vi "Dresden R2R Sputter 03.02.2018 IY24.vi"() -> ()   [LabVIEW 2009] (continued)
              shift-right: [w14079] -> w14054
              shift-left: i16? 0 -> [w14080]
              n8824 = Add(x=w14081, y=w14080) -> (x+y=w14079)
            }
            n8825 = Number To Decimal String(number=w14054) -> (decimal integer string=w14049)  [unwired: 1 in]
            n8826 = String Length(string=w14049) -> (length=w14050)
            n8827 = case shown="0, Default" w14050 {
              tunnel: w14049 -> [_ w14074 w14077 w14078]
              tunnel: [data[5B] w14072 w14075 w14078] -> w14048
              frame #0 {
              }
              frame #1 {
                n8828 = Concatenate Strings("00" ("string"), w14074) -> (w14072)
              }
              frame #2 {
                n8829 = Concatenate Strings("0" ("string"), w14077) -> (w14075)
              }
              frame #3 {
              }
            }
            n8830 = Concatenate Strings(w14047, w14048, "\n") -> (w14044)
            n8831 = VISA Write(VISA resource name=w14043, write buffer=w14044, error in (no error)=w14042) -> (VISA resource name out=w14046, error out=w14045)  [unwired: 1 out]
            n8832 = stacked-sequence {
              tunnel: [w14070] -> w14041
              tunnel: w14046 -> [w14070]
              tunnel: [w14069] -> w14040
              tunnel: w14045 -> [w14069]
              frame #0 {
                n8833 = Wait (ms)(milliseconds to wait=i32? 100) -> ()  [unwired: 1 out]
              }
            }
          }
          frame #4 {
            # "Cheksum 3 haneli olmalı"
            # "Address"
            n8834 = Concatenate Strings("002" ("write buffer"), "10" ("string"), "026" ("string"), "03" ("string"), "001" ("string")) -> (w14089)
            n8835 = String To Byte Array(string=w14089) -> (unsigned byte array=w14094)
            n8836 = for {
              tunnel: w14094 -> [w14115] mode=indexing
              shift-right: [w14113] -> w14096
              shift-left: i16? 0 -> [w14114]
              n8837 = Add(x=w14115, y=w14114) -> (x+y=w14113)
            }
            n8838 = Number To Decimal String(number=w14096) -> (decimal integer string=w14091)  [unwired: 1 in]
            n8839 = String Length(string=w14091) -> (length=w14092)
            n8840 = case shown="0, Default" w14092 {
              tunnel: w14091 -> [_ w14108 w14111 w14112]
              tunnel: [data[5B] w14106 w14109 w14112] -> w14090
              frame #0 {
              }
              frame #1 {
                n8841 = Concatenate Strings("00" ("string"), w14108) -> (w14106)
              }
              frame #2 {
                n8842 = Concatenate Strings("0" ("string"), w14111) -> (w14109)
              }
              frame #3 {
              }
            }
            n8843 = Concatenate Strings(w14089, w14090, "\n") -> (w14086)
            n8844 = VISA Write(VISA resource name=w14085, write buffer=w14086, error in (no error)=w14084) -> (VISA resource name out=w14088, error out=w14087)  [unwired: 1 out]
            n8845 = stacked-sequence {
              tunnel: [w14104] -> w14083
              tunnel: w14088 -> [w14104]
              tunnel: [w14103] -> w14082
              tunnel: w14087 -> [w14103]
              frame #0 {
                n8846 = Wait (ms)(milliseconds to wait=i32? 100) -> ()  [unwired: 1 out]
              }
            }
          }
          frame #5 {
            # "Address"
            n8847 = Concatenate Strings("002" ("write buffer"), "10" ("string"), "026" ("string"), "03" ("string"), "000" ("string")) -> (w14123)
            n8848 = String To Byte Array(string=w14123) -> (unsigned byte array=w14128)
            n8849 = for {
              tunnel: w14128 -> [w14149] mode=indexing
              shift-right: [w14147] -> w14130
              shift-left: i16? 0 -> [w14148]
              n8850 = Add(x=w14149, y=w14148) -> (x+y=w14147)
            }
            n8851 = Number To Decimal String(number=w14130) -> (decimal integer string=w14125)  [unwired: 1 in]
            n8852 = String Length(string=w14125) -> (length=w14126)
            n8853 = case shown="0, Default" w14126 {
              tunnel: w14125 -> [_ w14142 w14145 w14146]
              tunnel: [data[5B] w14140 w14143 w14146] -> w14124
              frame #0 {
              }
              frame #1 {
                n8854 = Concatenate Strings("00" ("string"), w14142) -> (w14140)
              }
              frame #2 {
                n8855 = Concatenate Strings("0" ("string"), w14145) -> (w14143)
              }
              frame #3 {
              }
            }
            n8856 = Concatenate Strings(w14123, w14124, "\n") -> (w14120)
            n8857 = VISA Write(VISA resource name=w14119, write buffer=w14120, error in (no error)=w14118) -> (VISA resource name out=w14122, error out=w14121)  [unwired: 1 out]
            n8858 = stacked-sequence {
              tunnel: [w14138] -> w14117
              tunnel: w14122 -> [w14138]
              tunnel: [w14137] -> w14116
              tunnel: w14121 -> [w14137]
              frame #0 {
                n8859 = Wait (ms)(milliseconds to wait=i32? 100) -> ()  [unwired: 1 out]
              }
            }
          }
          frame #6 {
            # "Cheksum 3 haneli olmalı"
            # "Address"
            n8860 = Concatenate Strings("002" ("write buffer"), "10" ("string"), "023" ("string"), "06" ("string"), "111111" ("string")) -> (w14157)
            n8861 = String To Byte Array(string=w14157) -> (unsigned byte array=w14162)
            n8862 = for {
              tunnel: w14162 -> [w14183] mode=indexing
              shift-right: [w14181] -> w14164
              shift-left: i16? 0 -> [w14182]
              n8863 = Add(x=w14183, y=w14182) -> (x+y=w14181)
            }
            n8864 = Number To Decimal String(number=w14164) -> (decimal integer string=w14159)  [unwired: 1 in]
            n8865 = String Length(string=w14159) -> (length=w14160)
            n8866 = case shown="0, Default" w14160 {
              tunnel: w14159 -> [_ w14176 w14179 w14180]
              tunnel: [data[5B] w14174 w14177 w14180] -> w14158
              frame #0 {
              }
              frame #1 {
                n8867 = Concatenate Strings("00" ("string"), w14176) -> (w14174)
              }
              frame #2 {
                n8868 = Concatenate Strings("0" ("string"), w14179) -> (w14177)
              }
              frame #3 {
              }
            }
            n8869 = Concatenate Strings(w14157, w14158, "\n") -> (w14154)
            n8870 = VISA Write(VISA resource name=w14153, write buffer=w14154, error in (no error)=w14152) -> (VISA resource name out=w14156, error out=w14155)  [unwired: 1 out]
            n8871 = stacked-sequence {
              tunnel: [w14172] -> w14151
              tunnel: w14156 -> [w14172]
              tunnel: [w14171] -> w14150
              tunnel: w14155 -> [w14171]
              frame #0 {
                n8872 = Wait (ms)(milliseconds to wait=i32? 100) -> ()  [unwired: 1 out]
              }
            }
          }
          frame #7 {
            # "Cheksum 3 haneli olmalı"
            # "Address"
            n8873 = Concatenate Strings("002" ("write buffer"), "10" ("string"), "023" ("string"), "06" ("string"), "000000" ("string")) -> (w14191)
            n8874 = String To Byte Array(string=w14191) -> (unsigned byte array=w14196)
            n8875 = for {
              tunnel: w14196 -> [w14217] mode=indexing
              shift-right: [w14215] -> w14198
              shift-left: i16? 0 -> [w14216]
              n8876 = Add(x=w14217, y=w14216) -> (x+y=w14215)
            }
            n8877 = Number To Decimal String(number=w14198) -> (decimal integer string=w14193)  [unwired: 1 in]
            n8878 = String Length(string=w14193) -> (length=w14194)
            n8879 = case shown="0, Default" w14194 {
              tunnel: w14193 -> [_ w14210 w14213 w14214]
              tunnel: [data[5B] w14208 w14211 w14214] -> w14192
              frame #0 {
              }
              frame #1 {
                n8880 = Concatenate Strings("00" ("string"), w14210) -> (w14208)
              }
              frame #2 {
                n8881 = Concatenate Strings("0" ("string"), w14213) -> (w14211)
              }
              frame #3 {
              }
            }
            n8882 = Concatenate Strings(w14191, w14192, "\n") -> (w14188)
            n8883 = VISA Write(VISA resource name=w14187, write buffer=w14188, error in (no error)=w14186) -> (VISA resource name out=w14190, error out=w14189)  [unwired: 1 out]
            n8884 = stacked-sequence {
              tunnel: [w14206] -> w14185
              tunnel: w14190 -> [w14206]
              tunnel: [w14205] -> w14184
              tunnel: w14189 -> [w14205]
              frame #0 {
                n8885 = Wait (ms)(milliseconds to wait=i32? 100) -> ()  [unwired: 1 out]
              }
            }
          }
        }
      }
      frame #2 {
        n8886 = Or(x="Set_speed Tp3", y="Tp3_auto_set_speed") -> (x .or. y?=w14241)
        n8887 = Compound Arithmetic op=OR("Start Tp3", "Tp_start_ch3_gui", "Tp3_auto_start") -> (w14223)
        n8888 = Compound Arithmetic op=OR("Stop Tp3", "Tp_stop_ch3_gui", "Tp3_auto_stop") -> (w14226)
        n8889 = Or(x="Low_speed Tp3", y="Tp3_auto_low_speed") -> (x .or. y?=w14224)
        n8890 = Or(x="Normal_speed Tp3", y="Tp3_auto_normal_speed") -> (x .or. y?=w14236)
        n8891 = case shown="False" w14223 {
          tunnel: [i16? 0 w14248] -> w14222
          frame #0 {
          }
          frame #1 {
            n8892 = local read "Ch3_Tp_start_safety"() -> (w14249)
            n8893 = case shown="True" w14249 {
              tunnel: [i16? 0 T/1] -> w14248
              frame #0 {
                n8894 = local write "Tp3_auto_start"(i16? 0 ("Tp1_auto_start")) -> ()
                n8895 = local write "Error Message"("TP can not be started.\nReason:\n*MP can not be open                           *TP-BV can not be open.       *Pressure difference                                between chamber and pipeline \nnot suitable.\n                                      \n" ("Error Message")) -> ()
              }
              frame #1 {
              }
            }
          }
        }
        n8896 = Build Array(i16? 0, w14222, w14226, w14241, w14224, w14236, "Start_initial Tp3", "Stop_initial Tp3", "Adress set") -> (w14233)
        n8897 = Boolean Array To Number(Boolean array=w14233) -> (number=w14246)
        n8898 = Mantissa & Exponent(0:w14246) -> (2:w14245)  [unwired: 1 out]
        n8899 = case shown="0, Default" w14245 {
          tunnel: w14221 -> [w14256 w14369 w14405 w14446 w14488 w14522 w14556 w14590]
          tunnel: w14220 -> [w14257 w14368 w14404 w14445 w14487 w14521 w14555 w14589]
          tunnel: [w14255 w14366 w14401 w14437 w14486 w14520 w14554 w14588] -> w14219
          tunnel: [w14254 w14365 w14400 w14436 w14485 w14519 w14553 w14587] -> w14218
          frame #0 {
            n8900 = stacked-sequence {
              tunnel: w14256 -> [w14273 _]
              tunnel: w14257 -> [w14272 _]
              tunnel: [_ w14324] -> w14255
              tunnel: [_ w14323] -> w14254
              frame #0 {
                # "Address"
                # "Cheksum 3 haneli olmalı"
                # "Address"
                n8901 = Concatenate Strings("003" ("write buffer"), "00" ("string"), "309" ("string"), "02" ("string"), "=?" ("string")) -> (w14282)
                n8902 = String To Byte Array(string=w14282) -> (unsigned byte array=w14287)
                n8903 = for {
                  tunnel: w14287 -> [w14319] mode=indexing
                  shift-right: [w14317] -> w14289
                  shift-left: i16? 0 -> [w14318]
                  n8904 = Add(x=w14319, y=w14318) -> (x+y=w14317)
                }
                n8905 = Number To Decimal String(number=w14289) -> (decimal integer string=w14284)  [unwired: 1 in]
                n8906 = String Length(string=w14284) -> (length=w14285)
                n8907 = case shown="0, Default" w14285 {
                  tunnel: w14284 -> [_ w14312 w14315 w14316]
                  tunnel: [data[5B] w14310 w14313 w14316] -> w14283
                  frame #0 {
                  }
                  frame #1 {
                    n8908 = Concatenate Strings("00" ("string"), w14312) -> (w14310)
                  }
                  frame #2 {
                    n8909 = Concatenate Strings("0" ("string"), w14315) -> (w14313)
                  }
                  frame #3 {
                  }
                }
                n8910 = Concatenate Strings(w14282, w14283, "\n") -> (w14274)
                n8911 = VISA Write(VISA resource name=w14273, write buffer=w14274, error in (no error)=w14272) -> (VISA resource name out=w14277, error out=w14276)  [unwired: 1 out]
                n8912 = stacked-sequence {
                  tunnel: [w14308] -> w14279
                  tunnel: w14277 -> [w14308]
                  tunnel: [w14307] -> w14278
                  tunnel: w14276 -> [w14307]
                  frame #0 {
                    n8913 = Wait (ms)(milliseconds to wait=i32? 100) -> ()  [unwired: 1 out]
                  }
                }
                n8914 = property class="Instr"(reference=w14279, error in=w14278) -> (reference out=w14281, error out=w14280, "Serial Settings:Number of Bytes at Serial Port"=w14275)
                n8915 = VISA Read(VISA resource name=w14281, byte count=w14275, error in (no error)=w14280) -> (VISA resource name out=w14263, read buffer=w14270, error out=w14262)  [unwired: 1 out]
                "Read_data 6" <- w14270
                n8916 = String Length(string=w14270) -> (length=w14271)
                n8917 = Not Equal To 0?(x=w14271) -> (x != 0?=w14261)
                n8918 = feedback #279() -> (w14258)  [unwired: 1 in]
                n8919 = Concatenate Strings("003" ("regular expression"), "1030906" ("regular expression")) -> (w14269)
                n8920 = Match Pattern(string=w14270, regular expression=w14269) -> (after substring=w14264)  [unwired: 4 out]
                n8921 = case shown="True" w14261 {
                  tunnel: [i16? 0 w14299] -> w14260
                  tunnel: [T/1 i16? 0] -> w14259
                  tunnel: w14258 -> [_ w14297]
                  frame #0 {
                  }
                  frame #1 {
                    n8922 = call "Elapsed Time133"(2:w14297) -> (16:w14300)  [unwired: 11 in, 7 out]
                    n8923 = Greater?(x=w14300, y=dbl? 5.0) -> (0:w14299)
                  }
                }
                "Com_ok 3" <- w14260
                n8924 = String Length(string=w14264) -> (length=w14266)
                n8925 = Not Equal To 0?(x=w14266) -> (x != 0?=w14265)
                n8926 = case shown="True" w14265 {
                  tunnel: w14264 -> [_ w14303]
                  frame #0 {
                  }
                  frame #1 {
                    n8927 = String Subset(string=w14303, length (rest)=i32? 6 ("length (rest)")) -> (substring=w14304)  [unwired: 1 out]
                    n8928 = Decimal String To Number(string=w14304) -> (number=→"Tp3_speed_gui" →"Turbo_pump_speed 5")  [unwired: 3 out]
                  }
                }
              }
              frame #1 {
                # "Address"
                # "Cheksum 3 haneli olmalı"
                # "Address"
                n8929 = Concatenate Strings("003" ("write buffer"), "00" ("string"), "307" ("string"), "02" ("string"), "=?" ("string")) -> (w14337)
                n8930 = String To Byte Array(string=w14337) -> (unsigned byte array=w14342)
                n8931 = for {
                  tunnel: w14342 -> [w14363] mode=indexing
                  shift-right: [w14361] -> w14344
                  shift-left: i16? 0 -> [w14362]
                  n8932 = Add(x=w14363, y=w14362) -> (x+y=w14361)
                }
                n8933 = Number To Decimal String(number=w14344) -> (decimal integer string=w14339)  [unwired: 1 in]
                n8934 = String Length(string=w14339) -> (length=w14340)
                n8935 = case shown="0, Default" w14340 {
                  tunnel: w14339 -> [_ w14356 w14359 w14360]
                  tunnel: [data[5B] w14354 w14357 w14360] -> w14338
                  frame #0 {
                  }
                  frame #1 {
                    n8936 = Concatenate Strings("00" ("string"), w14356) -> (w14354)
                  }
                  frame #2 {
                    n8937 = Concatenate Strings("0" ("string"), w14359) -> (w14357)
                  }
                  frame #3 {
                  }
                }
                n8938 = Concatenate Strings(w14337, w14338, "\n") -> (w14329)
                n8939 = VISA Write(VISA resource name=w14321, write buffer=w14329, error in (no error)=w14322) -> (VISA resource name out=w14332, error out=w14331)  [unwired: 1 out]
                n8940 = stacked-sequence {
                  tunnel: [w14352] -> w14334
                  tunnel: w14332 -> [w14352]
                  tunnel: [w14351] -> w14333
                  tunnel: w14331 -> [w14351]
                  frame #0 {
                    n8941 = Wait (ms)(milliseconds to wait=i32? 100) -> ()  [unwired: 1 out]
                  }
                }
                n8942 = property class="Instr"(reference=w14334, error in=w14333) -> (reference out=w14336, error out=w14335, "Serial Settings:Number of Bytes at Serial Port"=w14330)
                n8943 = VISA Read(VISA resource name=w14336, byte count=w14330, error in (no error)=w14335) -> (VISA resource name out=w14324, read buffer=w14328, error out=w14323)  [unwired: 1 out]
                "Read_data 7" <- w14328
                n8944 = Concatenate Strings("003" ("regular expression"), "1030706" ("regular expression")) -> (w14327)
                n8945 = Match Pattern(string=w14328, regular expression=w14327) -> (after substring=→"after substring 3")  [unwired: 4 out]
              }
            }
          }
          frame #1 {
            # "Address"
            n8946 = Concatenate Strings("003" ("write buffer"), "10" ("string"), "010" ("string"), "06" ("string"), "111111" ("string")) -> (w14373)
            n8947 = String To Byte Array(string=w14373) -> (unsigned byte array=w14378)
            n8948 = for {
              tunnel: w14378 -> [w14399] mode=indexing
              shift-right: [w14397] -> w14380
              shift-left: i16? 0 -> [w14398]
              n8949 = Add(x=w14399, y=w14398) -> (x+y=w14397)
            }
            n8950 = Number To Decimal String(number=w14380) -> (decimal integer string=w14375)  [unwired: 1 in]
            n8951 = String Length(string=w14375) -> (length=w14376)
            n8952 = local write "Tp3_auto_start"(i16? 0 ("Tp3_auto_start")) -> ()
            n8953 = case shown="0, Default" w14376 {
              tunnel: w14375 -> [_ w14392 w14395 w14396]
              tunnel: [data[5B] w14390 w14393 w14396] -> w14374
              frame #0 {
              }
              frame #1 {
                n8954 = Concatenate Strings("00" ("string"), w14392) -> (w14390)
              }
              frame #2 {
                n8955 = Concatenate Strings("0" ("string"), w14395) -> (w14393)
              }
              frame #3 {
              }
            }
            n8956 = local write "Tp3_stop_cmnd"(i16? 0 ("Tp3_auto_start")) -> ()
            n8957 = Concatenate Strings(w14373, w14374, "\n") -> (w14370)
            n8958 = VISA Write(VISA resource name=w14369, write buffer=w14370, error in (no error)=w14368) -> (VISA resource name out=w14372, error out=w14371)  [unwired: 1 out]
            n8959 = stacked-sequence {
              tunnel: [w14388] -> w14366
              tunnel: w14372 -> [w14388]
              tunnel: [w14387] -> w14365
              tunnel: w14371 -> [w14387]
              frame #0 {
                n8960 = Wait (ms)(milliseconds to wait=i32? 100) -> ()  [unwired: 1 out]
              }
            }
          }
          frame #2 {
            # "Cheksum 3 haneli olmalı"
            # "Address"
            n8961 = Concatenate Strings("003" ("write buffer"), "10" ("string"), "010" ("string"), "06" ("string"), "000000" ("string")) -> (w14409)
            n8962 = String To Byte Array(string=w14409) -> (unsigned byte array=w14414)
            n8963 = for {
              tunnel: w14414 -> [w14435] mode=indexing
              shift-right: [w14433] -> w14416
              shift-left: i16? 0 -> [w14434]
              n8964 = Add(x=w14435, y=w14434) -> (x+y=w14433)
            }
            n8965 = Number To Decimal String(number=w14416) -> (decimal integer string=w14411)  [unwired: 1 in]
            n8966 = local write "Tp3_auto_stop"(i16? 0 ("Tp3_auto_stop")) -> ()
            n8967 = String Length(string=w14411) -> (length=w14412)
            n8968 = case shown="0, Default" w14412 {
              tunnel: w14411 -> [_ w14428 w14431 w14432]
              tunnel: [data[5B] w14426 w14429 w14432] -> w14410
              frame #0 {
              }
              frame #1 {
                n8969 = Concatenate Strings("00" ("string"), w14428) -> (w14426)
              }
              frame #2 {
                n8970 = Concatenate Strings("0" ("string"), w14431) -> (w14429)
              }
              frame #3 {
              }
            }
            n8971 = Concatenate Strings(w14409, w14410, "\n") -> (w14406)
            n8972 = VISA Write(VISA resource name=w14405, write buffer=w14406, error in (no error)=w14404) -> (VISA resource name out=w14408, error out=w14407)  [unwired: 1 out]
            n8973 = stacked-sequence {
              tunnel: [w14424] -> w14401
              tunnel: w14408 -> [w14424]
              tunnel: [w14423] -> w14400
              tunnel: w14407 -> [w14423]
              frame #0 {
                n8974 = Wait (ms)(milliseconds to wait=i32? 100) -> ()  [unwired: 1 out]
              }
            }
            "Tp3_stop_cmnd" <- T/1 ("Tp3_stop_cmnd")
          }
          frame #3 {
            # "Cheksum 3 haneli olmalı"
            # "Address"
            n8975 = Multiply(x="Low_speed_value 3", y=data[16B]) -> (x*y=w14442)
            n8976 = To Unsigned Long Integer(number=w14442) -> (unsigned 32bit integer=w14441)
            n8977 = Number To Decimal String(number=w14441) -> (decimal integer string=w14439)  [unwired: 1 out]
            n8978 = String Length(string=w14439) -> (length=w14440)
            n8979 = case shown="0, Default" w14440 {
              tunnel: w14439 -> [_ w14466 w14469 w14470]
              tunnel: [data[5B] w14465 w14468 w14470] -> w14438
              frame #0 {
              }
              frame #1 {
                n8980 = Concatenate Strings(w14466, "00" ("string")) -> (w14465)
              }
              frame #2 {
                n8981 = Concatenate Strings(w14469, "0" ("string")) -> (w14468)
              }
              frame #3 {
              }
            }
            n8982 = Concatenate Strings("003" ("write buffer"), "10" ("string"), "707" ("string"), "06" ("string"), "00" ("string"), w14438) -> (w14450)
            n8983 = String To Byte Array(string=w14450) -> (unsigned byte array=w14455)
            n8984 = for {
              tunnel: w14455 -> [w14484] mode=indexing
              shift-right: [w14482] -> w14457
              shift-left: i16? 0 -> [w14483]
              n8985 = Add(x=w14484, y=w14483) -> (x+y=w14482)
            }
            n8986 = Number To Decimal String(number=w14457) -> (decimal integer string=w14452)  [unwired: 1 in]
            n8987 = String Length(string=w14452) -> (length=w14453)
            n8988 = case shown="0, Default" w14453 {
              tunnel: w14452 -> [_ w14477 w14480 w14481]
              tunnel: [data[5B] w14475 w14478 w14481] -> w14451
              frame #0 {
              }
              frame #1 {
                n8989 = Concatenate Strings("00" ("string"), w14477) -> (w14475)
              }
              frame #2 {
                n8990 = Concatenate Strings("0" ("string"), w14480) -> (w14478)
              }
              frame #3 {
              }
            }
            n8991 = Concatenate Strings(w14450, w14451, "\n") -> (w14447)
            n8992 = VISA Write(VISA resource name=w14446, write buffer=w14447, error in (no error)=w14445) -> (VISA resource name out=w14449, error out=w14448)  [unwired: 1 out]
            n8993 = stacked-sequence {
              tunnel: [w14473] -> w14437
              tunnel: w14449 -> [w14473]
              tunnel: [w14472] -> w14436
              tunnel: w14448 -> [w14472]
              frame #0 {
                n8994 = Wait (ms)(milliseconds to wait=i32? 100) -> ()  [unwired: 1 out]
              }
            }
          }
          frame #4 {
            # "Cheksum 3 haneli olmalı"
            # "Address"
            n8995 = Concatenate Strings("003" ("write buffer"), "10" ("string"), "026" ("string"), "03" ("string"), "001" ("string")) -> (w14492)
            n8996 = String To Byte Array(string=w14492) -> (unsigned byte array=w14497)
            n8997 = for {
              tunnel: w14497 -> [w14518] mode=indexing
              shift-right: [w14516] -> w14499
              shift-left: i16? 0 -> [w14517]
              n8998 = Add(x=w14518, y=w14517) -> (x+y=w14516)
            }
            n8999 = Number To Decimal String(number=w14499) -> (decimal integer string=w14494)  [unwired: 1 in]
            n9000 = String Length(string=w14494) -> (length=w14495)
            n9001 = case shown="0, Default" w14495 {
              tunnel: w14494 -> [_ w14511 w14514 w14515]
              tunnel: [data[5B] w14509 w14512 w14515] -> w14493
              frame #0 {
              }
              frame #1 {
                n9002 = Concatenate Strings("00" ("string"), w14511) -> (w14509)
              }
              frame #2 {
                n9003 = Concatenate Strings("0" ("string"), w14514) -> (w14512)
              }
              frame #3 {
              }
            }
            n9004 = Concatenate Strings(w14492, w14493, "\n") -> (w14489)
            n9005 = VISA Write(VISA resource name=w14488, write buffer=w14489, error in (no error)=w14487) -> (VISA resource name out=w14491, error out=w14490)  [unwired: 1 out]
            n9006 = stacked-sequence {
              tunnel: [w14507] -> w14486
              tunnel: w14491 -> [w14507]
              tunnel: [w14506] -> w14485
              tunnel: w14490 -> [w14506]
              frame #0 {
                n9007 = Wait (ms)(milliseconds to wait=i32? 100) -> ()  [unwired: 1 out]
              }
            }
          }
          frame #5 {
            # "Cheksum 3 haneli olmalı"
            # "Address"
            n9008 = Concatenate Strings("003" ("write buffer"), "10" ("string"), "026" ("string"), "03" ("string"), "000" ("string")) -> (w14526)
            n9009 = String To Byte Array(string=w14526) -> (unsigned byte array=w14531)
            n9010 = for {
              tunnel: w14531 -> [w14552] mode=indexing
              shift-right: [w14550] -> w14533
              shift-left: i16? 0 -> [w14551]
              n9011 = Add(x=w14552, y=w14551) -> (x+y=w14550)
            }
            n9012 = Number To Decimal String(number=w14533) -> (decimal integer string=w14528)  [unwired: 1 in]
            n9013 = String Length(string=w14528) -> (length=w14529)
            n9014 = case shown="0, Default" w14529 {
              tunnel: w14528 -> [_ w14545 w14548 w14549]
              tunnel: [data[5B] w14543 w14546 w14549] -> w14527
              frame #0 {
              }
              frame #1 {
                n9015 = Concatenate Strings("00" ("string"), w14545) -> (w14543)
              }
              frame #2 {
                n9016 = Concatenate Strings("0" ("string"), w14548) -> (w14546)
              }
              frame #3 {
              }
            }
            n9017 = Concatenate Strings(w14526, w14527, "\n") -> (w14523)
            n9018 = VISA Write(VISA resource name=w14522, write buffer=w14523, error in (no error)=w14521) -> (VISA resource name out=w14525, error out=w14524)  [unwired: 1 out]
            n9019 = stacked-sequence {
              tunnel: [w14541] -> w14520
              tunnel: w14525 -> [w14541]
              tunnel: [w14540] -> w14519
              tunnel: w14524 -> [w14540]
              frame #0 {
                n9020 = Wait (ms)(milliseconds to wait=i32? 100) -> ()  [unwired: 1 out]
              }
            }
          }
          frame #6 {
            # "Cheksum 3 haneli olmalı"
            # "Address"
            n9021 = Concatenate Strings("003" ("write buffer"), "10" ("string"), "023" ("string"), "06" ("string"), "111111" ("string")) -> (w14560)
            n9022 = String To Byte Array(string=w14560) -> (unsigned byte array=w14565)
            n9023 = for {
              tunnel: w14565 -> [w14586] mode=indexing
              shift-right: [w14584] -> w14567
              shift-left: i16? 0 -> [w14585]
              n9024 = Add(x=w14586, y=w14585) -> (x+y=w14584)
            }
            n9025 = Number To Decimal String(number=w14567) -> (decimal integer string=w14562)  [unwired: 1 in]
            n9026 = String Length(string=w14562) -> (length=w14563)
            n9027 = case shown="0, Default" w14563 {
              tunnel: w14562 -> [_ w14579 w14582 w14583]
              tunnel: [data[5B] w14577 w14580 w14583] -> w14561
              frame #0 {
              }
              frame #1 {
                n9028 = Concatenate Strings("00" ("string"), w14579) -> (w14577)
              }
              frame #2 {
                n9029 = Concatenate Strings("0" ("string"), w14582) -> (w14580)
              }
              frame #3 {
              }
            }
            n9030 = Concatenate Strings(w14560, w14561, "\n") -> (w14557)
            n9031 = VISA Write(VISA resource name=w14556, write buffer=w14557, error in (no error)=w14555) -> (VISA resource name out=w14559, error out=w14558)  [unwired: 1 out]
            n9032 = stacked-sequence {
              tunnel: [w14575] -> w14554
              tunnel: w14559 -> [w14575]
              tunnel: [w14574] -> w14553
              tunnel: w14558 -> [w14574]
              frame #0 {
                n9033 = Wait (ms)(milliseconds to wait=i32? 100) -> ()  [unwired: 1 out]
              }
            }
          }
          frame #7 {
            # "Cheksum 3 haneli olmalı"
            # "Address"
            n9034 = Concatenate Strings("003" ("write buffer"), "10" ("string"), "023" ("string"), "06" ("string"), "000000" ("string")) -> (w14594)
            n9035 = String To Byte Array(string=w14594) -> (unsigned byte array=w14599)
            n9036 = for {
              tunnel: w14599 -> [w14620] mode=indexing
              shift-right: [w14618] -> w14601
              shift-left: i16? 0 -> [w14619]
              n9037 = Add(x=w14620, y=w14619) -> (x+y=w14618)
            }
            n9038 = Number To Decimal String(number=w14601) -> (decimal integer string=w14596)  [unwired: 1 in]
            n9039 = String Length(string=w14596) -> (length=w14597)
            n9040 = case shown="0, Default" w14597 {
              tunnel: w14596 -> [_ w14613 w14616 w14617]
              tunnel: [data[5B] w14611 w14614 w14617] -> w14595
              frame #0 {
              }
              frame #1 {
                n9041 = Concatenate Strings("00" ("string"), w14613) -> (w14611)
              }
              frame #2 {
                n9042 = Concatenate Strings("0" ("string"), w14616) -> (w14614)
              }
              frame #3 {
              }
            }
            n9043 = Concatenate Strings(w14594, w14595, "\n") -> (w14591)
            n9044 = VISA Write(VISA resource name=w14590, write buffer=w14591, error in (no error)=w14589) -> (VISA resource name out=w14593, error out=w14592)  [unwired: 1 out]
            n9045 = stacked-sequence {
              tunnel: [w14609] -> w14588
              tunnel: w14593 -> [w14609]
              tunnel: [w14608] -> w14587
              tunnel: w14592 -> [w14608]
              frame #0 {
                n9046 = Wait (ms)(milliseconds to wait=i32? 100) -> ()  [unwired: 1 out]
              }
            }
          }
        }
      }
      frame #3 {
        n9047 = Or(x="Tp4_low_speed", y="Tp4_auto_low_speed") -> (x .or. y?=w14635)
        n9048 = Or(x="Tp4_set_speed", y="Tp4_auto_set_speed") -> (x .or. y?=w14638)
        n9049 = Or(x="Tp4_normal_speed", y="Tp4_auto_normal_speed") -> (x .or. y?=w14632)
        n9050 = Compound Arithmetic op=OR("Tp4_stop", "Tp_stop_ch4_gui", "Tp4_auto_stop") -> (w14623)
        n9051 = Compound Arithmetic op=OR("Tp4_start", "Tp_start_ch4_gui", "Tp4_auto_start") -> (w14622)
        n9052 = case shown="True" w14622 {
          tunnel: [i16? 0 w14650] -> w14621
          frame #0 {
          }
          frame #1 {
            n9053 = local read "Ch4_Tp_start_safety"() -> (w14651)
            n9054 = case shown="True" w14651 {
              tunnel: [i16? 0 T/1] -> w14650
              frame #0 {
                n9055 = local write "Tp4_auto_start"(i16? 0 ("Tp1_auto_start")) -> ()
                n9056 = local write "Error Message"("TP can not be started.\nReason:\n*MP can not be open. \n    *TP-BV can not be open.\n *Pressure difference between\nchamber and pipeline \nnot suitable.\n" ("Error Message")) -> ()
              }
              frame #1 {
              }
            }
          }
        }
        n9057 = Build Array(i16? 0, w14621, w14623, w14638, w14635, w14632, "Start_initial Tp4", "Stop_initial Tp4") -> (w14642)
        n9058 = Boolean Array To Number(Boolean array=w14642) -> (number=w14648)
        n9059 = Mantissa & Exponent(0:w14648) -> (2:w14647)  [unwired: 1 out]
        n9060 = case shown="0, Default" w14647 {
          tunnel: w14646 -> [w14656 w14771 w14807 w14848 w14890 w14924 w14958 w14992]
          tunnel: w14645 -> [w14657 w14770 w14806 w14847 w14889 w14923 w14957 w14991]
          tunnel: [w14659 w14769 w14805 w14846 w14888 w14922 w14956 w14990] -> w14644
          tunnel: [w14658 w14768 w14804 w14845 w14887 w14921 w14955 w14989] -> w14643
          frame #0 {
            n9061 = stacked-sequence {
              tunnel: w14656 -> [w14675 _]
              tunnel: w14657 -> [w14674 _]
              tunnel: [_ w14726] -> w14659
              tunnel: [_ w14725] -> w14658
              frame #0 {
                # "Address"
                # "Cheksum 3 haneli olmalı"
                # "Address"
                n9062 = Concatenate Strings("004" ("write buffer"), "00" ("string"), "309" ("string"), "02" ("string"), "=?" ("string")) -> (w14684)
                n9063 = String To Byte Array(string=w14684) -> (unsigned byte array=w14689)
                n9064 = for {
                  tunnel: w14689 -> [w14721] mode=indexing
                  shift-right: [w14719] -> w14691
                  shift-left: i16? 0 -> [w14720]
                  n9065 = Add(x=w14721, y=w14720) -> (x+y=w14719)
                }
                n9066 = Number To Decimal String(number=w14691) -> (decimal integer string=w14686)  [unwired: 1 in]
                n9067 = String Length(string=w14686) -> (length=w14687)
                n9068 = case shown="0, Default" w14687 {
                  tunnel: w14686 -> [_ w14714 w14717 w14718]
                  tunnel: [data[5B] w14712 w14715 w14718] -> w14685
                  frame #0 {
                  }
                  frame #1 {
                    n9069 = Concatenate Strings("00" ("string"), w14714) -> (w14712)
                  }
                  frame #2 {
                    n9070 = Concatenate Strings("0" ("string"), w14717) -> (w14715)
                  }
                  frame #3 {
                  }
                }
                n9071 = Concatenate Strings(w14684, w14685, "\n") -> (w14676)
                n9072 = VISA Write(VISA resource name=w14675, write buffer=w14676, error in (no error)=w14674) -> (VISA resource name out=w14679, error out=w14678)  [unwired: 1 out]
                n9073 = stacked-sequence {
                  tunnel: [w14710] -> w14681
                  tunnel: w14679 -> [w14710]
                  tunnel: [w14709] -> w14680
                  tunnel: w14678 -> [w14709]
                  frame #0 {
                    n9074 = Wait (ms)(milliseconds to wait=i32? 100) -> ()  [unwired: 1 out]
                  }
                }
                n9075 = property class="Instr"(reference=w14681, error in=w14680) -> (reference out=w14683, error out=w14682, "Serial Settings:Number of Bytes at Serial Port"=w14677)
                n9076 = VISA Read(VISA resource name=w14683, byte count=w14677, error in (no error)=w14682) -> (VISA resource name out=w14665, read buffer=w14672, error out=w14664)  [unwired: 1 out]
                "Read_data 8" <- w14672
                n9077 = String Length(string=w14672) -> (length=w14673)
                n9078 = Not Equal To 0?(x=w14673) -> (x != 0?=w14660)
                n9079 = Concatenate Strings("004" ("regular expression"), "1030906" ("regular expression")) -> (w14671)
                n9080 = feedback #280() -> (w14662)  [unwired: 1 in]
                n9081 = Match Pattern(string=w14672, regular expression=w14671) -> (after substring=w14666)  [unwired: 4 out]
                n9082 = case shown="True" w14660 {
                  tunnel: [i16? 0 w14701] -> w14661
                  tunnel: [T/1 i16? 0] -> w14663
                  tunnel: w14662 -> [_ w14699]
                  frame #0 {
                  }
                  frame #1 {
                    n9083 = call "Elapsed Time134"(2:w14699) -> (16:w14702)  [unwired: 11 in, 7 out]
                    n9084 = Greater?(x=w14702, y=dbl? 5.0) -> (0:w14701)
                  }
                }
                "Com_ok 4" <- w14661
                n9085 = String Length(string=w14666) -> (length=w14668)
                n9086 = Not Equal To 0?(x=w14668) -> (x != 0?=w14667)
                n9087 = case shown="True" w14667 {
                  tunnel: w14666 -> [_ w14705]
                  frame #0 {
                  }
                  frame #1 {
                    n9088 = String Subset(string=w14705, length (rest)=i32? 6 ("length (rest)")) -> (substring=w14706)  [unwired: 1 out]
                    n9089 = Decimal String To Number(string=w14706) -> (number=→"Turbo_pump_speed 4" →"Tp4_speed_gui")  [unwired: 3 out]
                  }
                }
              }
              frame #1 {
                # "Address"
                # "Cheksum 3 haneli olmalı"
                # "Address"
                n9090 = Concatenate Strings("004" ("write buffer"), "00" ("string"), "307" ("string"), "02" ("string"), "=?" ("string")) -> (w14739)
                n9091 = String To Byte Array(string=w14739) -> (unsigned byte array=w14744)
                n9092 = for {
                  tunnel: w14744 -> [w14765] mode=indexing
                  shift-right: [w14763] -> w14746
                  shift-left: i16? 0 -> [w14764]
                  n9093 = Add(x=w14765, y=w14764) -> (x+y=w14763)
                }
                n9094 = Number To Decimal String(number=w14746) -> (decimal integer string=w14741)  [unwired: 1 in]
                n9095 = String Length(string=w14741) -> (length=w14742)
                n9096 = case shown="0, Default" w14742 {
                  tunnel: w14741 -> [_ w14758 w14761 w14762]
                  tunnel: [data[5B] w14756 w14759 w14762] -> w14740
                  frame #0 {
                  }
                  frame #1 {
                    n9097 = Concatenate Strings("00" ("string"), w14758) -> (w14756)
                  }
                  frame #2 {
                    n9098 = Concatenate Strings("0" ("string"), w14761) -> (w14759)
                  }
                  frame #3 {
                  }
                }
                n9099 = Concatenate Strings(w14739, w14740, "\n") -> (w14731)
                n9100 = VISA Write(VISA resource name=w14723, write buffer=w14731, error in (no error)=w14724) -> (VISA resource name out=w14734, error out=w14733)  [unwired: 1 out]
                n9101 = stacked-sequence {
                  tunnel: [w14754] -> w14736
                  tunnel: w14734 -> [w14754]
                  tunnel: [w14753] -> w14735
                  tunnel: w14733 -> [w14753]
                  frame #0 {
                    n9102 = Wait (ms)(milliseconds to wait=i32? 100) -> ()  [unwired: 1 out]
                  }
                }
                n9103 = property class="Instr"(reference=w14736, error in=w14735) -> (reference out=w14738, error out=w14737, "Serial Settings:Number of Bytes at Serial Port"=w14732)
                n9104 = VISA Read(VISA resource name=w14738, byte count=w14732, error in (no error)=w14737) -> (VISA resource name out=w14726, read buffer=w14730, error out=w14725)  [unwired: 1 out]
                "Read_data 9" <- w14730
                n9105 = Concatenate Strings("004" ("regular expression"), "1030706" ("regular expression")) -> (w14729)
                n9106 = Match Pattern(string=w14730, regular expression=w14729) -> (after substring=→"after substring 4")  [unwired: 4 out]
              }
            }
          }
          frame #1 {
            # "Cheksum 3 haneli olmalı"
            # "Address"
            n9107 = Concatenate Strings("004" ("write buffer"), "10" ("string"), "010" ("string"), "06" ("string"), "111111" ("string")) -> (w14775)
            n9108 = String To Byte Array(string=w14775) -> (unsigned byte array=w14780)
            n9109 = for {
              tunnel: w14780 -> [w14801] mode=indexing
              shift-right: [w14799] -> w14782
              shift-left: i16? 0 -> [w14800]
              n9110 = Add(x=w14801, y=w14800) -> (x+y=w14799)
            }
            n9111 = local write "Tp4_auto_start"(i16? 0 ("Tp4_auto_start")) -> ()
            n9112 = Number To Decimal String(number=w14782) -> (decimal integer string=w14777)  [unwired: 1 in]
            n9113 = String Length(string=w14777) -> (length=w14778)
            n9114 = case shown="0, Default" w14778 {
              tunnel: w14777 -> [_ w14794 w14797 w14798]
              tunnel: [data[5B] w14792 w14795 w14798] -> w14776
              frame #0 {
              }
              frame #1 {
                n9115 = Concatenate Strings("00" ("string"), w14794) -> (w14792)
              }
              frame #2 {
                n9116 = Concatenate Strings("0" ("string"), w14797) -> (w14795)
              }
              frame #3 {
              }
            }
            n9117 = local write "Tp4_stop_cmnd"(i16? 0 ("Tp4_stop_cmnd")) -> ()
            n9118 = Concatenate Strings(w14775, w14776, "\n") -> (w14772)
            n9119 = VISA Write(VISA resource name=w14771, write buffer=w14772, error in (no error)=w14770) -> (VISA resource name out=w14774, error out=w14773)  [unwired: 1 out]
            n9120 = stacked-sequence {
              tunnel: [w14790] -> w14769
              tunnel: w14774 -> [w14790]
              tunnel: [w14789] -> w14768
              tunnel: w14773 -> [w14789]
              frame #0 {
                n9121 = Wait (ms)(milliseconds to wait=i32? 100) -> ()  [unwired: 1 out]
              }
            }
          }
          frame #2 {
            # "Cheksum 3 haneli olmalı"
            # "Address"
            n9122 = Concatenate Strings("004" ("write buffer"), "10" ("string"), "010" ("string"), "06" ("string"), "000000" ("string")) -> (w14811)
            n9123 = String To Byte Array(string=w14811) -> (unsigned byte array=w14816)
            n9124 = for {
              tunnel: w14816 -> [w14837] mode=indexing
              shift-right: [w14835] -> w14818
              shift-left: i16? 0 -> [w14836]
              n9125 = Add(x=w14837, y=w14836) -> (x+y=w14835)
            }
            n9126 = local write "Tp4_auto_stop"(i16? 0 ("Tp4_auto_stop")) -> ()
            n9127 = Number To Decimal String(number=w14818) -> (decimal integer string=w14813)  [unwired: 1 in]
            n9128 = String Length(string=w14813) -> (length=w14814)
            n9129 = case shown="0, Default" w14814 {
              tunnel: w14813 -> [_ w14830 w14833 w14834]
              tunnel: [data[5B] w14828 w14831 w14834] -> w14812
              frame #0 {
              }
              frame #1 {
                n9130 = Concatenate Strings("00" ("string"), w14830) -> (w14828)
              }
              frame #2 {
                n9131 = Concatenate Strings("0" ("string"), w14833) -> (w14831)
              }
              frame #3 {
              }
            }
            n9132 = Concatenate Strings(w14811, w14812, "\n") -> (w14808)
            n9133 = VISA Write(VISA resource name=w14807, write buffer=w14808, error in (no error)=w14806) -> (VISA resource name out=w14810, error out=w14809)  [unwired: 1 out]
            n9134 = stacked-sequence {
              tunnel: [w14826] -> w14805
              tunnel: w14810 -> [w14826]
              tunnel: [w14825] -> w14804
              tunnel: w14809 -> [w14825]